vi "UHR-Fleezers Control (host) - 12.0(oscillate_test).vi"() -> ()   [LabVIEW 2014] (continued)
                                }
                                frame #3 {
                                n428 = Wait (ms)(milliseconds to wait=u32 500) -> ()  [unwired: 1 out]
                                }
                                frame #4 {
                                n429 = property on="Trap Raster Scan" class="Bool (strict)"("Val(Sgnl)"=TRUE ("Value (Signaling)")) -> ()  [unwired: 2 in, 2 out]
                                }
                                frame #5 {
                                n430 = Wait (ms)(milliseconds to wait=u32 2000) -> ()  [unwired: 1 out]
                                }
                                frame #6 {
                                n431 = flat-sequence {
                                tunnel: w713 -> [w720]
                                frame #0 {
                                n432 = while {
                                stop <- w716 stop-if-true
                                n433 = local read "Raster Scanning..."() -> (w715:bool)
                                n434 = local read "Saving..."() -> (w718:bool)
                                n435 = Wait (ms)(milliseconds to wait=u32 100) -> ()  [unwired: 1 out]
                                n436 = Not(x=w718) -> (.not. x?=w717:bool)
                                n437 = Not(x=w715) -> (.not. x?=w714:bool)
                                n438 = And(x=w717, y=w714) -> (x .and. y?=w716:bool)
                                }
                                }
                                frame #1 {
                                n439 = local read "Tether"() -> (w721:bool)
                                n440 = case shown="True" w721 {
                                tunnel: w720 -> [_ w723]
                                frame False {
                                n441 = property on="Fish" class="Bool (strict)"("Val(Sgnl)"="Fish again after \nraster break?") -> ()  [unwired: 2 in, 2 out]
                                }
                                frame True {
                                n442 = stacked-sequence {
                                tunnel: w723 -> [_ w727 _ _ _ _ _ _]
                                frame #0 {
                                n443 = property on="Trap D (MHz)" class="DigNum (strict)"("Val(Sgnl)"="Move to D 2 (MHz)") -> ()  [unwired: 2 in, 2 out]
                                n444 = case shown="True" "Flow ON after\ntether testing?" {
                                frame False {
                                }
                                frame True {
                                n445 = property on="Sample Channel\nFlow" class="Bool (strict)"("Val(Sgnl)"=TRUE ("Value (Signaling)")) -> ()  [unwired: 2 in, 2 out]
                                }
                                }
                                }
                                frame #1 {
                                n446 = flat-sequence {
                                tunnel: w727 -> [w728]
                                frame #0 {
                                n447 = case shown="\"6\"" w728 {
                                frame Default {
                                }
                                frame "6" {
                                n448 = flat-sequence {
                                frame #0 {
                                n449 = Wait (ms)(milliseconds to wait=u32 500) -> ()  [unwired: 1 out]
                                }
                                frame #1 {
                                n450 = property on="Green ON/Interlacing" class="Bool (strict)"("Val(Sgnl)"=TRUE ("Green Laser ON/Interlacing")) -> ()  [unwired: 2 in, 2 out]
                                }
                                }
                                }
                                }
                                }
                                frame #1 {
                                n451 = case shown="True" "Save at end (5, 6)" {
                                selector: "Save at end (5, 6)" -> [_ w732]
                                frame False {
                                }
                                frame True {
                                n452 = flat-sequence {
                                tunnel: w732 -> [w734]
                                frame #0 {
                                n453 = Wait (ms)(milliseconds to wait=u32 500) -> ()  [unwired: 1 out]
                                }
                                frame #1 {
                                n454 = local write "Start Saving"(w734) -> ()
                                }
                                }
                                }
                                }
                                }
                                }
                                }
                                frame #2 {
                                n455 = local read "Bead Sep. Int. Time (s)"() -> (w737:dbl)
                                n456 = Multiply(x=w737, y=1000.0) -> (x*y=w736:dbl)
                                n457 = Wait (ms)(milliseconds to wait=w736) -> ()  [unwired: 1 out]
                                }
                                frame #3 {
                                n458 = property on="Remove Offset" class="Bool (strict)"("Val(Sgnl)"=TRUE ("Value (Signaling)")) -> ()  [unwired: 2 in, 2 out]
                                }
                                frame #4 {
                                n459 = property on="Read FX file" class="Bool (strict)"("Val(Sgnl)"=TRUE ("Value (Signaling)")) -> ()  [unwired: 2 in, 2 out]
                                }
                                frame #5 {
                                n460 = Wait (ms)(milliseconds to wait=u32 300) -> ()  [unwired: 1 out]
                                }
                                frame #6 {
                                n461 = local read "Bad fit error"() -> (w746:dbl)
                                n462 = local read "Fit offset"() -> (w749:dbl)
                                n463 = Greater Or Equal?(x=w746, y="Bad fit thresh") -> (x >= y?=→"Bad fit":bool)
                                n464 = Greater Or Equal?(x=w749, y="Fit offset thresh") -> (x >= y?=→"Multiple tether":bool)
                                n465 = local read "Hyst. error"() -> (w743:dbl)
                                n466 = Greater Or Equal?(x=w743, y="Hysteresis thresh") -> (x >= y?=→"Hysteresis":bool)
                                }
                                frame #7 {
                                w754 = 0
                                n467 = local read "Bad fit error"() -> (w756:dbl)
                                n468 = local read "Hyst. error"() -> (w755:dbl)
                                n469 = local read "Fit offset"() -> (w757:dbl)
                                n470 = local read "Multiple tether"() -> (w763:bool)
                                n471 = local read "Hysteresis"() -> (w761:bool)
                                n472 = local read "Bad fit"() -> (w762:bool)
                                n473 = Not(x=w761) -> (.not. x?=w753:bool)
                                n474 = Not(x=w762) -> (.not. x?=w759:bool)
                                n475 = Greater?(x=w757, y=w754) -> (0:w752:bool)
                                n476 = Greater?(x=w756, y=w754) -> (0:w751:bool)
                                n477 = Greater?(x=w755, y=w754) -> (0:w750:bool)
                                n478 = Not(x=w763) -> (.not. x?=w760:bool)
                                n479 = Compound Arithmetic op=AND(w760, w759, w753, w752, w751, w750) -> (w758:bool)
                                "Good tether" <- w758
                                n480 = case shown="True" w758 {
                                frame False {
                                }
                                frame True {
                                n481 = call <vilib>:"Beep.vi"("use system alert? (T)"=FALSE, "duration (msec)"=u32 200, "frequency (Hz)"=u32 2000) -> ()  [unwired: 9 in]
                                }
                                }
                                }
                                }
                                }
                                }
                                }
                                }
                                }
                                }
                                }
                                frame "2", Default {
                                }
                              }
                            }
                            frame #3 {
                              n482 = local read "Multiple tether"() -> (w769:bool)
                              n483 = And(x="Break multiple", y=w769) -> (x .and. y?=w767:bool)
                              n484 = case shown="True" w767 {
                                frame False {
                                }
                                frame True {
                                n485 = stacked-sequence {
                                frame #0 {
                                n486 = property on="Trap D (MHz)" class="DigNum (strict)"("Val(Sgnl)"="Trap D to \nbreak (MHz)") -> ()  [unwired: 2 in, 2 out]
                                }
                                frame #1 {
                                n487 = case shown="True" "Fish after\nmultiple break" {
                                frame False {
                                }
                                frame True {
                                n488 = while {
                                stop <- w774 stop-if-true
                                n489 = local read "Multiple tether"() -> (w776:bool)
                                n490 = local read "Fish"() -> (w773:bool)
                                n491 = local read "Stop All"() -> (w772:bool)
                                n492 = Wait (ms)(milliseconds to wait=u32 100) -> ()  [unwired: 1 out]
                                n493 = Not(x=w776) -> (.not. x?=w775:bool)
                                n494 = Compound Arithmetic op=OR(w772, w775, w773) -> (w774:bool)
                                }
                                }
                                }
                                }
                                frame #2 {
                                n495 = local read "Fish after\nmultiple break"() -> (w781:bool)
                                n496 = local read "Stage Moving"() -> (w780:bool)
                                n497 = Not(x=w780) -> (.not. x?=w778:bool)
                                n498 = And(x=w781, y=w778) -> (x .and. y?=w779:bool)
                                n499 = property on="Fish" class="Bool (strict)"("Val(Sgnl)"=w779) -> ()  [unwired: 2 in, 2 out]
                                }
                                }
                                }
                              }
                            }
                            frame #4 {
                              n500 = local read "Bad fit"() -> (w783:bool)
                              n501 = And(x="Break bad fit", y=w783) -> (x .and. y?=w782:bool)
                              n502 = case shown="True" w782 {
                                frame False {
                                }
                                frame True {
                                n503 = stacked-sequence {
                                frame #0 {
                                n504 = local read "Trap D to \nbreak (MHz)"() -> (w785:dbl)
                                n505 = property on="Trap D (MHz)" class="DigNum (strict)"("Val(Sgnl)"=w785) -> ()  [unwired: 2 in, 2 out]
                                }
                                frame #1 {
                                n506 = case shown="True" "Fish after\nbad fit break?" {
                                frame False {
                                }
                                frame True {
                                n507 = while {
                                stop <- w789 stop-if-true
                                n508 = local read "Stop All"() -> (w787:bool)
                                n509 = local read "Bad fit"() -> (w788:bool)
                                n510 = local read "Fish"() -> (w790:bool)
                                n511 = Not(x=w788) -> (.not. x?=w791:bool)
                                n512 = Wait (ms)(milliseconds to wait=u32 100) -> ()  [unwired: 1 out]
                                n513 = Compound Arithmetic op=OR(w787, w791, w790) -> (w789:bool)
                                }
                                }
                                }
                                }
                                frame #2 {
                                n514 = local read "Fish after\nbad fit break?"() -> (w793:bool)
                                n515 = local read "Stage Moving"() -> (w796:bool)
                                n516 = Not(x=w796) -> (.not. x?=w795:bool)
                                n517 = And(x=w793, y=w795) -> (x .and. y?=w794:bool)
                                n518 = property on="Fish" class="Bool (strict)"("Val(Sgnl)"=w794) -> ()  [unwired: 2 in, 2 out]
                                }
                                }
                                }
                              }
                            }
                            frame #5 {
                              n519 = local read "Hysteresis"() -> (w798:bool)
                              n520 = And(x="Break hyst", y=w798) -> (x .and. y?=w797:bool)
                              n521 = case shown="True" w797 {
                                frame False {
                                }
                                frame True {
                                n522 = stacked-sequence {
                                frame #0 {
                                n523 = local read "Trap D to \nbreak (MHz)"() -> (w800:dbl)
                                n524 = property on="Trap D (MHz)" class="DigNum (strict)"("Val(Sgnl)"=w800) -> ()  [unwired: 2 in, 2 out]
                                }
                                frame #1 {
                                n525 = case shown="True" "Fish ater hyst?" {
                                frame False {
                                }
                                frame True {
                                n526 = while {
                                stop <- w806 stop-if-true
                                n527 = local read "Hysteresis"() -> (w805:bool)
                                n528 = local read "Stop All"() -> (w802:bool)
                                n529 = local read "Fish"() -> (w803:bool)
                                n530 = Wait (ms)(milliseconds to wait=u32 100) -> ()  [unwired: 1 out]
                                n531 = Not(x=w805) -> (.not. x?=w804:bool)
                                n532 = Compound Arithmetic op=OR(w802, w804, w803) -> (w806:bool)
                                }
                                }
                                }
                                }
                                frame #2 {
                                n533 = local read "Fish ater hyst?"() -> (w811:bool)
                                n534 = local read "Stage Moving"() -> (w810:bool)
                                n535 = Not(x=w810) -> (.not. x?=w809:bool)
                                n536 = And(x=w811, y=w809) -> (x .and. y?=w808:bool)
                                n537 = property on="Fish" class="Bool (strict)"("Val(Sgnl)"=w808) -> ()  [unwired: 2 in, 2 out]
                                }
                                }
                                }
                              }
                            }
                            frame #6 {
                              n538 = local read "Good tether"() -> (w812:bool)
                              n539 = case shown="True" w812 {
                                frame False {
                                }
                                frame True {
                                n540 = case shown="\"1\"" "If good, then:" {
                                frame "0", Default {
                                }
                                frame "1" {
                                n541 = property on="Force FB Script" class="Bool (strict)"("Val(Sgnl)"=TRUE ("Value (Signaling)")) -> ()  [unwired: 2 in, 2 out]
                                }
                                }
                                }
                              }
                            }
                          }
                        }
                        frame "7" {
                          n542 = property on="Force FB Script" class="Bool (strict)"("Val(Sgnl)"=TRUE ("Value (Signaling)")) -> ()  [unwired: 2 in, 2 out]
                        }
                        frame "8" {
                          n543 = property on="Fixed Traps Script" class="Bool (strict)"("Val(Sgnl)"=TRUE ("Value (Signaling)")) -> ()  [unwired: 2 in, 2 out]
                        }
                      }
                      "Tether" <- "Tether Alarm?"
                    }
                  }
                }
                frame #2 {
                  n544 = local read "Oscillate Set 1"() -> (w822:bool)
                  n545 = local read "Stop All"() -> (w820:bool)
                  n546 = Or(x=w822, y=w817) -> (x .or. y?=w819:bool)
                  n547 = Not(x=w819) -> (.not. x?=w821:bool)
                  n548 = Compound Arithmetic op=OR(w820, w821) -> (w818:bool)
                }
              }
              n549 = node-c288() -> ()  [unwired: 2 out]
            }
            n550 = node-c288(w572) -> ()  [unwired: 1 out]
          }
        }
      }
      event "Fl. Triggered...": Value Change {
        n551 = event-data() -> ()  [unwired: 7 out]
        n552 = case shown="True" "Fl. Triggered..." {
          frame False {
          }
          frame True {
            n553 = node-c288() -> (w833:T26)  [unwired: 4 out]
            n554 = timed-loop {
              timing: w833 -> [_]
              timing-out: [_] -> w832
              tunnel: "Action" -> [w841]
              shift-right: [w838] -> _
              shift-left: u8 255 -> [w840]
              shift-right: [w835] -> _
              shift-left: 255 -> [w837]
              stop <- w834 stop-if-true
              # "Reset confocal spot"
              n555 = node-c288() -> ()  [unwired: 2 out]
              n556 = flat-sequence {
                tunnel: w841 -> [w861]
                tunnel: w840 -> [w860]
                tunnel: [w859] -> w839
                tunnel: w837 -> [w846]
                tunnel: [w845] -> w836
                tunnel: [w1245] -> w834
                tunnel: w839 -> [w1244]
                tunnel: [w1244] -> w838
                tunnel: [w1243] -> w835
                tunnel: w836 -> [w1243]
                frame #0 {
                  n557 = local read "Delta Fl. 2"() -> (w858:dbl)
                  n558 = local read "Delta Fl. 1"() -> (w853:dbl)
                  n559 = Multiply(x="Fl. D Thresh. (kHz)", y=1000.0) -> (x*y=w848:dbl)
                  n560 = Select(t=w853, s="APD to Watch", f=w858) -> (s? t:f=w849:dbl)
                  n561 = Greater?(x=w849, y=w848) -> (0:w854:bool)
                  n562 = Or(x="Force Yank", y=w854) -> (x .or. y?=w852:bool)
                  n563 = And(x=w852, y="Yank when?") -> (x .and. y?=w850:bool)
                  n564 = case shown="False" w850 {
                    tunnel: w861 -> [w864 w1067]
                    tunnel: w860 -> [w866 w1063]
                    tunnel: [w866 w1061] -> w859
                    tunnel: w849 -> [w872 _]
                    tunnel: w848 -> [w871 _]
                    tunnel: "Force Yank" -> [w869 _]
                    tunnel: w846 -> [w868 w1060]
                    tunnel: [w867 w1060] -> w845
                    frame False {
                      n565 = Negate(x=w871) -> (-x=w863:dbl)
                      n566 = local write "Fl. High"(TRUE ("Fl. High")) -> ()
                      n567 = Less?(x=w872, y=w863) -> (x < y?=w870:bool)
                      n568 = Or(x=w869, y=w870) -> (x .or. y?=w865:bool)
                      n569 = case shown="True" w865 {
                        tunnel: w868 -> [w873 w883]
                        tunnel: [w873 w882] -> w867
                        tunnel: w864 -> [_ w881]
                        frame False {
                        }
                        frame True {
                          n570 = flat-sequence {
                            tunnel: w883 -> [w889]
                            tunnel: w881 -> [w886]
                            tunnel: [w888] -> w880
                            tunnel: [w887] -> w879
                            tunnel: [w886] -> w878
                            tunnel: w877 -> [w885]
                            tunnel: [w885] -> w876
                            tunnel: w875 -> [w884]
                            tunnel: [w884] -> w874
                            tunnel: [w961] -> w882
                            tunnel: w880 -> [w961]
                            tunnel: w879 -> [w960]
                            tunnel: w878 -> [w959]
                            tunnel: w876 -> [w958]
                            tunnel: w874 -> [w957]
                            frame #0 {
                              n571 = call <vilib>:"Beep.vi"() -> ()  [unwired: 12 in]
                              n572 = local write "Waiting"(FALSE ("Waiting")) -> ()
                              n573 = Increment(x=w889) -> (x+1=w888:i32)
                              n574 = case shown="\"Yank\"" w886 {
                                tunnel: w888 -> [_ w894 _]
                                frame "Alarm", Default {
                                }
                                frame "Yank" {
                                n575 = flat-sequence {
                                tunnel: w894 -> [w897]
                                tunnel: [w896] -> w893
                                tunnel: [w895] -> w892
                                tunnel: w893 -> [w907]
                                tunnel: w892 -> [w908]
                                frame #0 {
                                n576 = local read "Yank Delay (s)"() -> (w900:dbl)
                                n577 = local read "N Array El"() -> (w895:u8)
                                n578 = Quotient & Remainder(x=w897, y=w895) -> (x-y*floor(x/y)=w896:i32)  [unwired: 1 out]
                                n579 = Multiply(x=w900, y=1000.0) -> (x*y=w898:dbl)
                                n580 = Wait (ms)(milliseconds to wait=w898) -> ()  [unwired: 1 out]
                                }
                                frame #1 {
                                n581 = local read "Yank to which?"() -> (w902:bool)
                                n582 = local read "Random Choice"() -> (w912:bool)
                                n583 = local read "Yank to Trap D (MHz)"() -> (w905:dbl[])
                                n584 = local read "Yank to SP"() -> (w906:dbl[])
                                n585 = Random Number (0-1)() -> (number: 0 to 1=w911:dbl)
                                n586 = Multiply(x=w908, y=w911) -> (x*y=w910:dbl)
                                n587 = Round Toward -Infinity(1:w910) -> (0:w909:dbl)
                                n588 = Select(t=w909, s=w912, f=w907) -> (s? t:f=w903:dbl)
                                n589 = Select(t=w905, s=w902, f=w906) -> (s? t:f=w904:dbl[])
                                n590 = Index Array(array=w904, index=w903) -> (element=w901:dbl)
                                n591 = case shown="False" w902 {
                                tunnel: w901 -> [w913 w941]
                                frame False {
                                n592 = flat-sequence {
                                tunnel: w913 -> [w914]
                                frame #0 {
                                n593 = property on="Trap Pos FB SP" class="DigNum (strict)"("Val(Sgnl)"=w914) -> ()  [unwired: 2 in, 2 out]
                                }
                                frame #1 {
                                n594 = Wait (ms)(milliseconds to wait=u32 700) -> ()  [unwired: 1 out]
                                }
                                frame #2 {
                                n595 = local read "Action (%)"() -> (w919:dbl)
                                n596 = Absolute Value(x=w919) -> (abs(x)=w918:dbl)
                                n597 = Greater?(x=w918, y=70.0) -> (0:w916:bool)
                                n598 = property on="Remove Action Offset" class="Bool (strict)"("Val(Sgnl)"=w916) -> ()  [unwired: 2 in, 2 out]
                                }
                                frame #3 {
                                n599 = for {
                                N: 4 -> [_]
                                n600 = flat-sequence {
                                frame #0 {
                                n601 = Wait (ms)(milliseconds to wait=u32 500) -> ()  [unwired: 1 out]
                                }
                                frame #1 {
                                n602 = local read "Action (%)"() -> (w925:dbl)
                                n603 = Absolute Value(x=w925) -> (abs(x)=w924:dbl)
                                n604 = Greater?(x=w924, y=70.0) -> (0:w922:bool)
                                n605 = property on="Remove Action Offset" class="Bool (strict)"("Val(Sgnl)"=w922) -> ()  [unwired: 2 in, 2 out]
                                }
                                }
                                }
                                }
                                frame #4 {
                                n606 = Wait (ms)(milliseconds to wait=u32 500) -> ()  [unwired: 1 out]
                                }
                                frame #5 {
                                n607 = local read "Mean"() -> (w933:dbl)
                                n608 = Greater?(x=w933, y=11.0) -> (0:w927:bool)
                                n609 = Not(x=w927) -> (.not. x?=w928:bool)
                                n610 = And(x=w928, y="Shift confocal") -> (x .and. y?=w930:bool)
                                n611 = And(x=w927, y="Shift confocal") -> (x .and. y?=w931:bool)
                                n612 = case shown="True" w931 {
                                frame False {
                                }
                                frame True {
                                n613 = local read "Confocal Y 2 (V)"() -> (w937:dbl)
                                n614 = local read "Confocal X 2 (V)"() -> (w936:dbl)
                                n615 = property on="AO1" class="Slide (strict)"("Val(Sgnl)"=w937) -> ()  [unwired: 2 in, 2 out]
                                n616 = property on="AO2" class="Slide (strict)"("Val(Sgnl)"=w936) -> ()  [unwired: 2 in, 2 out]
                                }
                                }
                                n617 = case shown="True" w930 {
                                frame False {
                                }
                                frame True {
                                n618 = local read "Confocal Y 1 (V)"() -> (w935:dbl)
                                n619 = local read "Confocal X 1 (V)"() -> (w934:dbl)
                                n620 = property on="AO1" class="Slide (strict)"("Val(Sgnl)"=w935) -> ()  [unwired: 2 in, 2 out]
                                n621 = property on="AO2" class="Slide (strict)"("Val(Sgnl)"=w934) -> ()  [unwired: 2 in, 2 out]
                                }
                                }
                                }
                                frame #6 {
                                n622 = Wait (ms)(milliseconds to wait=u32 1500) -> ()  [unwired: 1 out]
                                }
                                frame #7 {
                                n623 = property on="Rem fb disp offset" class="Bool (strict)"("Val(Sgnl)"=TRUE ("Value (Signaling)")) -> ()  [unwired: 2 in, 2 out]
                                n624 = property on="Remove Offset" class="Bool (strict)"("Val(Sgnl)"=TRUE ("Value (Signaling)")) -> ()  [unwired: 2 in, 2 out]
                                }
                                }
                                }
                                frame True {
                                n625 = flat-sequence {
                                tunnel: w941 -> [w942]
                                frame #0 {
                                n626 = property on="Trap D (MHz)" class="DigNum (strict)"("Val(Sgnl)"=w942) -> ()  [unwired: 2 in, 2 out]
                                }
                                frame #1 {
                                n627 = Wait (ms)(milliseconds to wait=u32 500) -> ()  [unwired: 1 out]
                                }
                                frame #2 {
                                n628 = local read "Shift confocal"() -> (w948:bool)
                                n629 = local read "Mean"() -> (w950:dbl)
                                n630 = Greater?(x=w950, y=11.0) -> (0:w947:bool)
                                n631 = Not(x=w947) -> (.not. x?=w946:bool)
                                n632 = And(x=w946, y=w948) -> (x .and. y?=w944:bool)
                                n633 = And(x=w947, y=w948) -> (x .and. y?=w945:bool)
                                n634 = case shown="True" w945 {
                                frame False {
                                }
                                frame True {
                                n635 = local read "Confocal Y 2 (V)"() -> (w954:dbl)
                                n636 = local read "Confocal X 2 (V)"() -> (w953:dbl)
                                n637 = property on="AO2" class="Slide (strict)"("Val(Sgnl)"=w953) -> ()  [unwired: 2 in, 2 out]
                                n638 = property on="AO1" class="Slide (strict)"("Val(Sgnl)"=w954) -> ()  [unwired: 2 in, 2 out]
                                }
                                }
                                n639 = case shown="True" w944 {
                                frame False {
                                }
                                frame True {
                                n640 = local read "Confocal X 1 (V)"() -> (w951:dbl)
                                n641 = local read "Confocal Y 1 (V)"() -> (w952:dbl)
                                n642 = property on="AO2" class="Slide (strict)"("Val(Sgnl)"=w951) -> ()  [unwired: 2 in, 2 out]
                                n643 = property on="AO1" class="Slide (strict)"("Val(Sgnl)"=w952) -> ()  [unwired: 2 in, 2 out]
                                }
                                }
                                }
                                }
                                }
                                }
                                }
                                }
                                }
                                frame "Image" {
                                n644 = property on="Confocal\nImage" class="Bool (strict)"("Val(Sgnl)"=TRUE ("Value (Signaling)")) -> ()  [unwired: 2 in, 2 out]
                                }
                              }
                              n645 = local write "Fl. High"(FALSE ("Fl. High")) -> ()
                              n646 = local read "Time (s)"() -> (w887:dbl)
                            }
                            frame #1 {
                              n647 = case shown="True" "Auto F Reset" {
                                tunnel: w960 -> [_ w965]
                                tunnel: w959 -> [_ w964]
                                tunnel: w958 -> [_ w963]
                                tunnel: w957 -> [_ w962]
                                frame False {
                                }
                                frame True {
                                n648 = node-c288() -> (w967:T26)  [unwired: 4 in]
                                n649 = timed-loop {
                                timing: w967 -> [_]
                                timing-out: [_] -> w966
                                tunnel: w965 -> [w972]
                                tunnel: w964 -> [w971]
                                tunnel: w963 -> [w970]
                                tunnel: w962 -> [w969]
                                stop <- w968 stop-if-true
                                n650 = node-c288() -> ()  [unwired: 1 in, 1 out]
                                n651 = local read "APD to Watch"() -> (w982:bool)
                                n652 = local read "Fl. D Thresh. (kHz)"() -> (w981:dbl)
                                n653 = local read "Delta Fl. 1"() -> (w983:dbl)
                                n654 = local read "Delta Fl. 2"() -> (w984:dbl)
                                n655 = local read "Fl. Triggered..."() -> (w975:bool)
                                n656 = local read "Stop All"() -> (w976:bool)
                                n657 = local read "Reset Force"() -> (w974:bool)
                                n658 = Multiply(x=w981, y=1000.0) -> (x*y=w979:dbl)
                                n659 = Not(x=w975) -> (.not. x?=w973:bool)
                                n660 = Select(t=w983, s=w982, f=w984) -> (s? t:f=w978:dbl)
                                n661 = Greater?(x=w978, y=w979) -> (0:w977:bool)
                                n662 = Compound Arithmetic op=OR(w977, w976, w973, w974) -> (w968:bool)
                                n663 = case shown="True" w968 {
                                tunnel: w972 -> [_ w988]
                                tunnel: w971 -> [_ w992]
                                tunnel: w970 -> [_ w991]
                                tunnel: w969 -> [_ w990]
                                frame False {
                                }
                                frame True {
                                n664 = case shown="\"Yank\"" w992 {
                                tunnel: w991 -> [_ w1002]
                                tunnel: w990 -> [_ w1000]
                                frame "Image", Default {
                                }
                                frame "Yank" {
                                n665 = flat-sequence {
                                tunnel: [w1005] -> w1003
                                tunnel: w1002 -> [w1005]
                                tunnel: [w1004] -> w1001
                                tunnel: w1000 -> [w1004]
                                tunnel: w1003 -> [w1011]
                                tunnel: w1001 -> [w1009]
                                frame #0 {
                                n666 = local read "Yank Delay (s)"() -> (w1008:dbl)
                                n667 = Multiply(x=w1008, y=1000.0) -> (x*y=w1006:dbl)
                                n668 = Wait (ms)(milliseconds to wait=w1006) -> ()  [unwired: 1 out]
                                }
                                frame #1 {
                                n669 = local read "Yank to which?"() -> (w1010:bool)
                                n670 = case shown="False" w1010 {
                                tunnel: w1011 -> [_ w1040]
                                tunnel: w1009 -> [w1012 _]
                                frame False {
                                n671 = flat-sequence {
                                tunnel: w1012 -> [w1013]
                                frame #0 {
                                n672 = property on="Trap Pos FB SP" class="DigNum (strict)"("Val(Sgnl)"=w1013) -> ()  [unwired: 2 in, 2 out]
                                }
                                frame #1 {
                                n673 = Wait (ms)(milliseconds to wait=u32 700) -> ()  [unwired: 1 out]
                                }
                                frame #2 {
                                n674 = local read "Action (%)"() -> (w1018:dbl)
                                n675 = Absolute Value(x=w1018) -> (abs(x)=w1017:dbl)
                                n676 = Greater?(x=w1017, y=70.0) -> (0:w1015:bool)
                                n677 = property on="Remove Action Offset" class="Bool (strict)"("Val(Sgnl)"=w1015) -> ()  [unwired: 2 in, 2 out]
                                }
                                frame #3 {
                                n678 = for {
                                N: 4 -> [_]
                                n679 = flat-sequence {
                                frame #0 {
                                n680 = Wait (ms)(milliseconds to wait=u32 500) -> ()  [unwired: 1 out]
                                }
                                frame #1 {
                                n681 = local read "Action (%)"() -> (w1024:dbl)
                                n682 = Absolute Value(x=w1024) -> (abs(x)=w1023:dbl)
                                n683 = Greater?(x=w1023, y=70.0) -> (0:w1021:bool)
                                n684 = property on="Remove Action Offset" class="Bool (strict)"("Val(Sgnl)"=w1021) -> ()  [unwired: 2 in, 2 out]
                                }
                                }
                                }
                                }
                                frame #4 {
                                n685 = Wait (ms)(milliseconds to wait=u32 500) -> ()  [unwired: 1 out]
                                }
                                frame #5 {
                                n686 = local read "Shift confocal"() -> (w1029:bool)
                                n687 = local read "Mean"() -> (w1032:dbl)
                                n688 = Greater?(x=w1032, y=11.0) -> (0:w1028:bool)
                                n689 = Not(x=w1028) -> (.not. x?=w1027:bool)
                                n690 = And(x=w1028, y=w1029) -> (x .and. y?=w1030:bool)
                                n691 = And(x=w1027, y=w1029) -> (x .and. y?=w1026:bool)
                                n692 = case shown="True" w1030 {
                                frame False {
                                }
                                frame True {
                                n693 = local read "Confocal X 2 (V)"() -> (w1035:dbl)
                                n694 = local read "Confocal Y 2 (V)"() -> (w1036:dbl)
                                n695 = property on="AO2" class="Slide (strict)"("Val(Sgnl)"=w1035) -> ()  [unwired: 2 in, 2 out]
                                n696 = property on="AO1" class="Slide (strict)"("Val(Sgnl)"=w1036) -> ()  [unwired: 2 in, 2 out]
                                }
                                }
                                n697 = case shown="True" w1026 {
                                frame False {
                                }
                                frame True {
                                n698 = local read "Confocal Y 1 (V)"() -> (w1034:dbl)
                                n699 = local read "Confocal X 1 (V)"() -> (w1033:dbl)
                                n700 = property on="AO1" class="Slide (strict)"("Val(Sgnl)"=w1034) -> ()  [unwired: 2 in, 2 out]
                                n701 = property on="AO2" class="Slide (strict)"("Val(Sgnl)"=w1033) -> ()  [unwired: 2 in, 2 out]
                                }
                                }
                                }
                                frame #6 {
                                n702 = Wait (ms)(milliseconds to wait=u32 1500) -> ()  [unwired: 1 out]
                                }
                                frame #7 {
                                n703 = property on="Remove Offset" class="Bool (strict)"("Val(Sgnl)"=TRUE ("Value (Signaling)")) -> ()  [unwired: 2 in, 2 out]
                                n704 = property on="Rem fb disp offset" class="Bool (strict)"("Val(Sgnl)"=TRUE ("Value (Signaling)")) -> ()  [unwired: 2 in, 2 out]
                                }
                                }
                                }
                                frame True {
                                n705 = flat-sequence {
                                tunnel: w1040 -> [w1041]
                                frame #0 {
                                n706 = property on="Trap D (MHz)" class="DigNum (strict)"("Val(Sgnl)"=w1041) -> ()  [unwired: 2 in, 2 out]
                                }
                                frame #1 {
                                n707 = Wait (ms)(milliseconds to wait=u32 500) -> ()  [unwired: 1 out]
                                }
                                frame #2 {
                                n708 = local read "Shift confocal"() -> (w1047:bool)
                                n709 = local read "Mean"() -> (w1048:dbl)
                                n710 = Greater?(x=w1048, y=11.0) -> (0:w1046:bool)
                                n711 = And(x=w1046, y=w1047) -> (x .and. y?=w1044:bool)
                                n712 = Not(x=w1046) -> (.not. x?=w1045:bool)
                                n713 = And(x=w1045, y=w1047) -> (x .and. y?=w1043:bool)
                                n714 = case shown="True" w1044 {
                                frame False {
                                }
                                frame True {
                                n715 = local read "Confocal Y 2 (V)"() -> (w1053:dbl)
                                n716 = local read "Confocal X 2 (V)"() -> (w1052:dbl)
                                n717 = property on="AO1" class="Slide (strict)"("Val(Sgnl)"=w1053) -> ()  [unwired: 2 in, 2 out]
                                n718 = property on="AO2" class="Slide (strict)"("Val(Sgnl)"=w1052) -> ()  [unwired: 2 in, 2 out]
                                }
                                }
                                n719 = case shown="True" w1043 {
                                frame False {
                                }
                                frame True {
                                n720 = local read "Confocal Y 1 (V)"() -> (w1051:dbl)
                                n721 = local read "Confocal X 1 (V)"() -> (w1050:dbl)
                                n722 = property on="AO2" class="Slide (strict)"("Val(Sgnl)"=w1050) -> ()  [unwired: 2 in, 2 out]
                                n723 = property on="AO1" class="Slide (strict)"("Val(Sgnl)"=w1051) -> ()  [unwired: 2 in, 2 out]
                                }
                                }
                                }
                                }
                                }
                                }
                                }
                                }
                                }
                                }
                                n724 = local read "Time (s)"() -> (w987:dbl)
                                n725 = Subtract(x=w988, y=w987) -> (x-y=w999:dbl)
                                n726 = Number To Decimal String(number=w999, width (-)=i16 0) -> (decimal integer string=w997:string)
                                n727 = Concatenate Strings(w997, " s fluorescence event") -> (w994:string)
                                n728 = local read "Messages"() -> (w995:string)
                                n729 = local write "Duration (s)"(w999) -> ()
                                n730 = call "Update messages.vi"("Message to add"=w994, "Old message string"=w995) -> ("New message string"=w993:string)
                                n731 = local write "Messages"(w993) -> ()
                                n732 = call <vilib>:"Beep.vi"() -> ()  [unwired: 12 in]
                                n733 = local write "Reset Force"(FALSE ("Force Reset")) -> ()
                                n734 = local write "Fl. High"(TRUE ("Fl. High")) -> ()
                                n735 = local write "Waiting"(TRUE ("Waiting")) -> ()
                                }
                                }
                                n736 = node-c288() -> ()  [unwired: 1 in, 1 out]
                                }
                                n737 = node-c288(w966) -> ()  [unwired: 1 out]
                                }
                              }
                            }
                          }
                          n738 = local read "Trap Pos FB SP"() -> (w875:fxp<+/-,16,1>)
                          n739 = local read "Trap D (MHz)"() -> (w877:dbl)
                        }
                      }
                    }
                    frame True {
                      n740 = flat-sequence {
                        tunnel: w1064 -> [w1074]
                        tunnel: [w1074] -> w1068
                        tunnel: w1067 -> [w1073]
                        tunnel: [w1073] -> w1066
                        tunnel: [w1072] -> w1065
                        tunnel: w1063 -> [w1071]
                        tunnel: [w1070] -> w1062
                        tunnel: w1059 -> [w1069]
                        tunnel: [w1069] -> w1058
                        tunnel: w1068 -> [w1146]
                        tunnel: w1066 -> [w1145]
                        tunnel: w1065 -> [w1144]
                        tunnel: w1062 -> [w1143]
                        tunnel: w1058 -> [w1142]
                        tunnel: [w1143] -> w1061
                        frame #0 {
                          n741 = call <vilib>:"Beep.vi"() -> ()  [unwired: 3 in, 9 out]
                          n742 = local write "Waiting"(FALSE ("Waiting")) -> ()
                          n743 = Increment(x=w1071) -> (x+1=w1070:u8)
                          n744 = case shown="\"Image\"" w1073 {
                            tunnel: w1070 -> [_ _ w1080 _]
                            frame "Image" {
                              n745 = property on="Confocal\nImage" class="Bool (strict)"("Val(Sgnl)"=TRUE ("Value (Signaling)")) -> ()  [unwired: 2 in, 2 out]
                            }
                            frame "Alarm", Default {
                            }
                            frame "Yank" {
                              n746 = flat-sequence {
                                tunnel: w1080 -> [w1083]
                                tunnel: [w1082] -> w1079
                                tunnel: ["N Array El"] -> w1078
                                tunnel: w1079 -> [w1097]
                                tunnel: w1078 -> [w1093]
                                frame #0 {
                                n747 = Multiply(x="Yank Delay (s)", y=1000.0) -> (x*y=w1086:dbl)
                                n748 = Quotient & Remainder(x=w1083, y="N Array El") -> (x-y*floor(x/y)=w1082:u8)  [unwired: 1 out]
                                n749 = Wait (ms)(milliseconds to wait=w1086) -> ()  [unwired: 1 out]
                                }
                                frame #1 {
                                n750 = Random Number (0-1)() -> (number: 0 to 1=w1094:dbl)
                                n751 = Multiply(x=w1093, y=w1094) -> (x*y=w1092:dbl)
                                n752 = Round Toward -Infinity(1:w1092) -> (0:w1091:dbl)
                                n753 = Select(t=w1091, s="Random Choice", f=w1097) -> (s? t:f=w1095:dbl)
                                n754 = Select(t="Yank to Trap D (MHz)", s="Yank to which?", f="Yank to SP") -> (s? t:f=w1088:dbl[])
                                n755 = Index Array(array=w1088, index=w1095) -> (element=w1098:dbl)
                                n756 = case shown="False" "Yank to which?" {
                                tunnel: w1098 -> [w1099 w1126]
                                frame False {
                                n757 = flat-sequence {
                                tunnel: w1099 -> [w1100]
                                frame #0 {
                                n758 = property on="Trap Pos FB SP" class="DigNum (strict)"("Val(Sgnl)"=w1100) -> ()  [unwired: 2 in, 2 out]
                                }
                                frame #1 {
                                n759 = Wait (ms)(milliseconds to wait=u32 700) -> ()  [unwired: 1 out]
                                }
                                frame #2 {
                                n760 = local read "Action (%)"() -> (w1105:dbl)
                                n761 = Absolute Value(x=w1105) -> (abs(x)=w1104:dbl)
                                n762 = Greater?(x=w1104, y=70.0) -> (0:w1102:bool)
                                n763 = property on="Remove Action Offset" class="Bool (strict)"("Val(Sgnl)"=w1102) -> ()  [unwired: 2 in, 2 out]
                                }
                                frame #3 {
                                n764 = for {
                                N: 4 -> [_]
                                n765 = flat-sequence {
                                frame #0 {
                                n766 = Wait (ms)(milliseconds to wait=u32 500) -> ()  [unwired: 1 out]
                                }
                                frame #1 {
                                n767 = local read "Action (%)"() -> (w1111:dbl)
                                n768 = Absolute Value(x=w1111) -> (abs(x)=w1110:dbl)
                                n769 = Greater?(x=w1110, y=70.0) -> (0:w1108:bool)
                                n770 = property on="Remove Action Offset" class="Bool (strict)"("Val(Sgnl)"=w1108) -> ()  [unwired: 2 in, 2 out]
                                }
                                }
                                }
                                }
                                frame #4 {
                                n771 = local read "Shift confocal"() -> (w1115:bool)
                                n772 = local read "Mean"() -> (w1118:dbl)
                                n773 = Greater?(x=w1118, y=11.0) -> (0:w1114:bool)
                                n774 = Not(x=w1114) -> (.not. x?=w1113:bool)
                                n775 = And(x=w1113, y=w1115) -> (x .and. y?=w1112:bool)
                                n776 = And(x=w1114, y=w1115) -> (x .and. y?=w1116:bool)
                                n777 = case shown="True" w1116 {
                                frame False {
                                }
                                frame True {
                                n778 = local read "Confocal X 2 (V)"() -> (w1121:dbl)
                                n779 = local read "Confocal Y 2 (V)"() -> (w1122:dbl)
                                n780 = property on="AO2" class="Slide (strict)"("Val(Sgnl)"=w1121) -> ()  [unwired: 2 in, 2 out]
                                n781 = property on="AO1" class="Slide (strict)"("Val(Sgnl)"=w1122) -> ()  [unwired: 2 in, 2 out]
                                }
                                }
                                n782 = case shown="True" w1112 {
                                frame False {
                                }
                                frame True {
                                n783 = local read "Confocal X 1 (V)"() -> (w1119:dbl)
                                n784 = local read "Confocal Y 1 (V)"() -> (w1120:dbl)
                                n785 = property on="AO1" class="Slide (strict)"("Val(Sgnl)"=w1120) -> ()  [unwired: 2 in, 2 out]
                                n786 = property on="AO2" class="Slide (strict)"("Val(Sgnl)"=w1119) -> ()  [unwired: 2 in, 2 out]
                                }
                                }
                                }
                                frame #5 {
                                n787 = Wait (ms)(milliseconds to wait=u32 1500) -> ()  [unwired: 1 out]
                                }
                                frame #6 {
                                n788 = property on="Remove Offset" class="Bool (strict)"("Val(Sgnl)"=TRUE ("Value (Signaling)")) -> ()  [unwired: 2 in, 2 out]
                                n789 = property on="Rem fb disp offset" class="Bool (strict)"("Val(Sgnl)"=TRUE ("Value (Signaling)")) -> ()  [unwired: 2 in, 2 out]
                                }
                                }
                                }
                                frame True {
                                n790 = flat-sequence {
                                tunnel: w1126 -> [w1127]
                                frame #0 {
                                n791 = property on="Trap D (MHz)" class="DigNum (strict)"("Val(Sgnl)"=w1127) -> ()  [unwired: 2 in, 2 out]
                                }
                                frame #1 {
                                n792 = Wait (ms)(milliseconds to wait=u32 500) -> ()  [unwired: 1 out]
                                }
                                frame #2 {
                                n793 = local read "Shift confocal"() -> (w1131:bool)
                                n794 = local read "Mean"() -> (w1129:dbl)
                                n795 = Greater?(x=w1129, y=11.0) -> (0:w1132:bool)
                                n796 = Not(x=w1132) -> (.not. x?=w1133:bool)
                                n797 = And(x=w1133, y=w1131) -> (x .and. y?=w1135:bool)
                                n798 = And(x=w1132, y=w1131) -> (x .and. y?=w1134:bool)
                                n799 = case shown="True" w1134 {
                                frame False {
                                }
                                frame True {
                                n800 = local read "Confocal Y 2 (V)"() -> (w1139:dbl)
                                n801 = local read "Confocal X 2 (V)"() -> (w1138:dbl)
                                n802 = property on="AO1" class="Slide (strict)"("Val(Sgnl)"=w1139) -> ()  [unwired: 2 in, 2 out]